vi "UHR-Fleezers Control (host) - 10.8MV_trial.vi"() -> ()   [LabVIEW 2010] (continued)
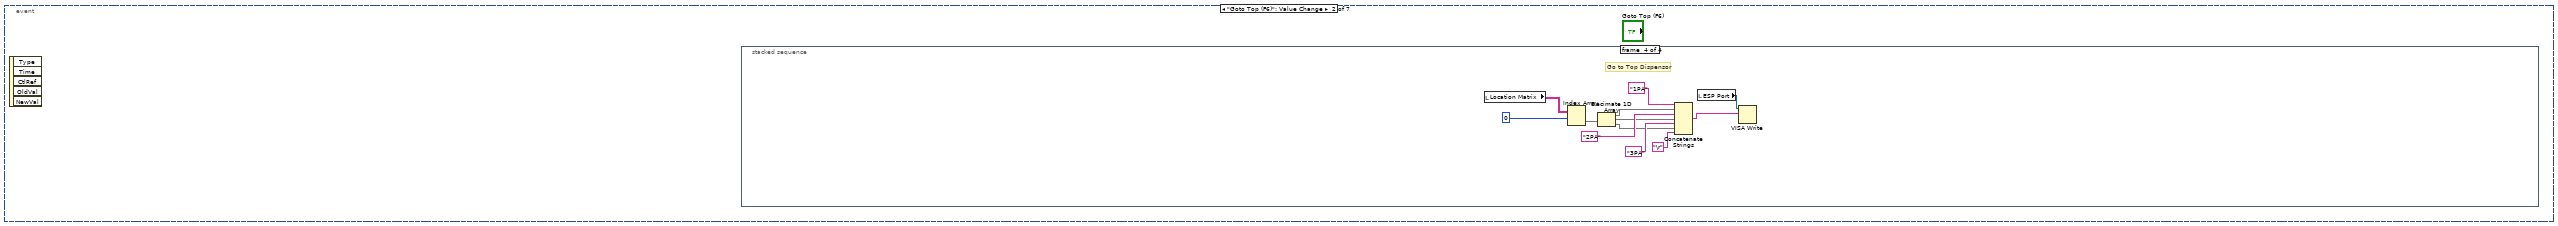
[diagram p3: hidden frame]
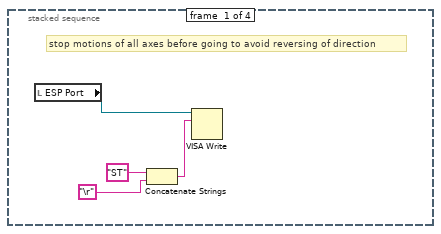
[diagram p4: hidden frame]
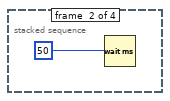
[diagram p5: hidden frame]
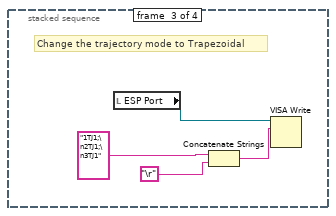
[diagram p6: hidden frame]
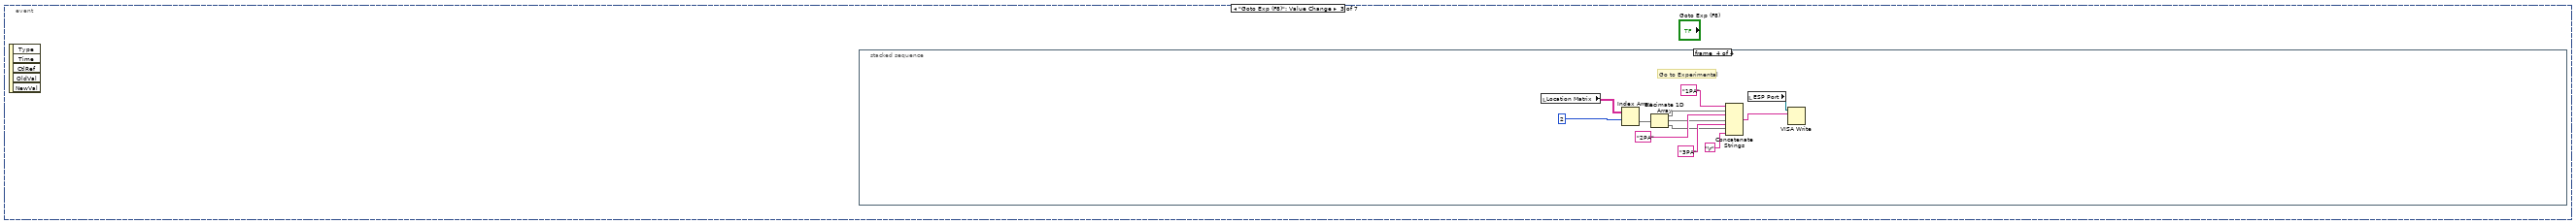
[diagram p7: hidden frame]
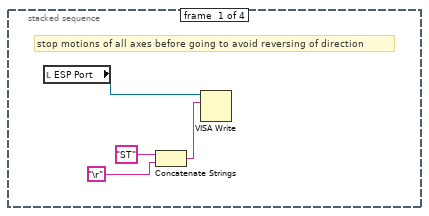
[diagram p8: hidden frame]
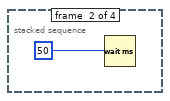
[diagram p9: hidden frame]
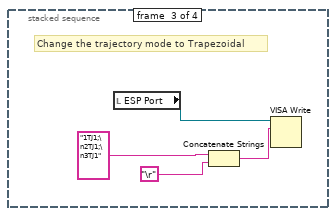
[diagram p10: hidden frame]
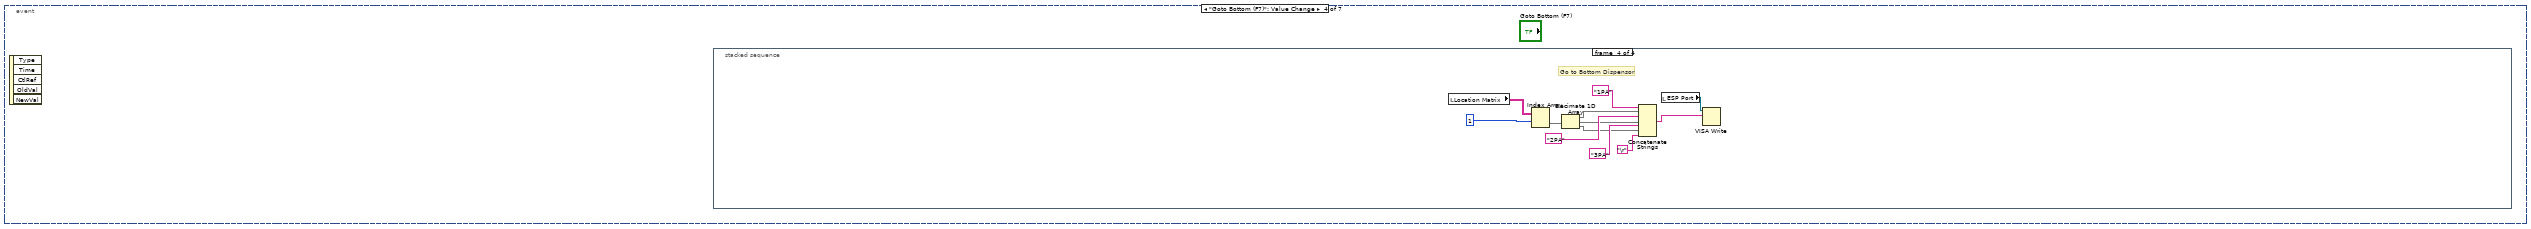
[diagram p11: hidden frame]
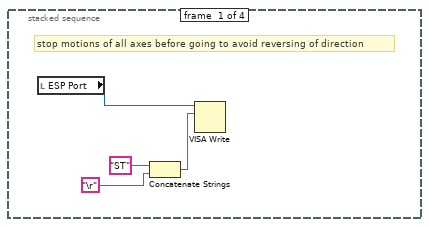
[diagram p12: hidden frame]
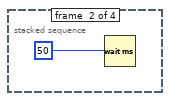
[diagram p13: hidden frame]
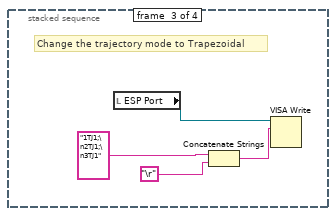
[diagram p14: hidden frame]
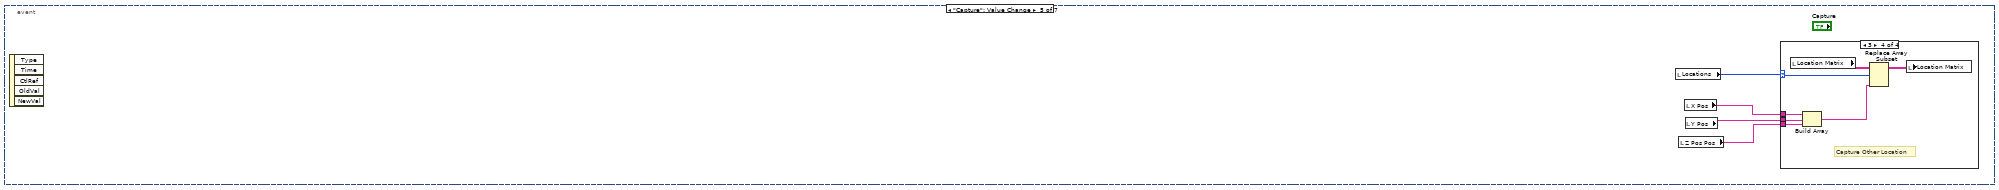
[diagram p15: hidden frame]
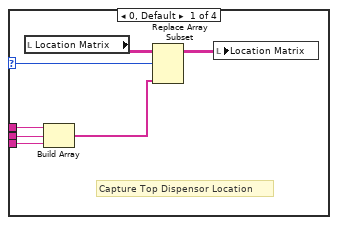
[diagram p16: hidden frame]
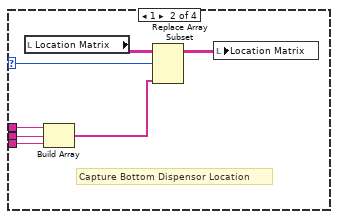
[diagram p17: hidden frame]
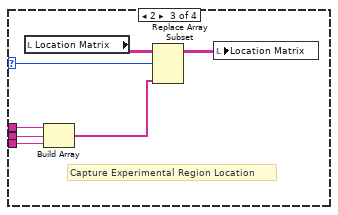
[diagram p18: hidden frame]
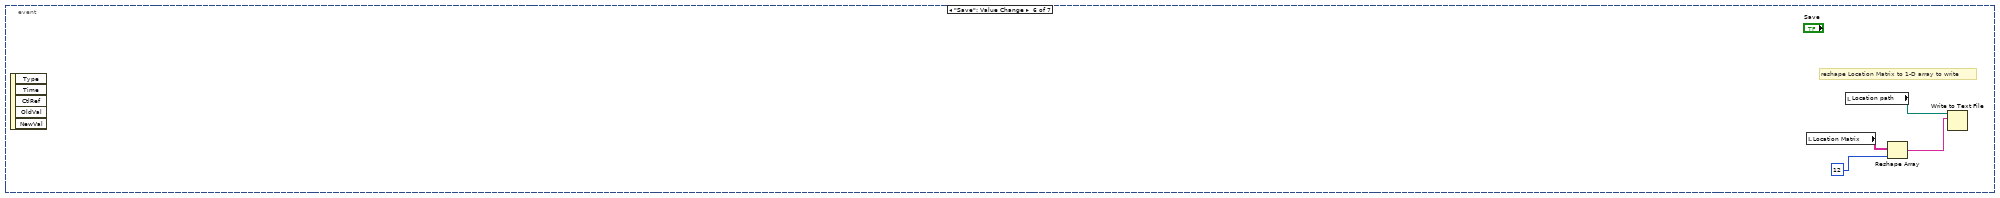
[diagram p19: hidden frame]
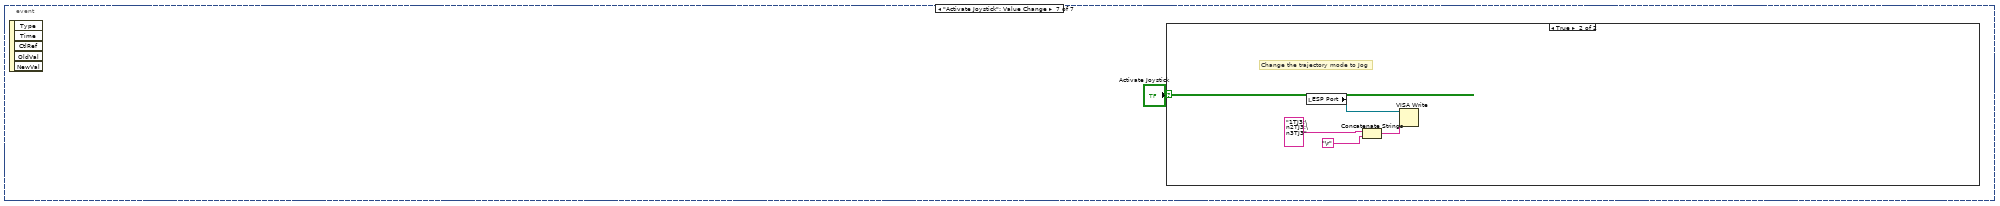
[diagram p20: hidden frame]
                  frame False {
                  }
                  frame True {
                    n1970 = Close File(refnum=w8541) -> ()  [unwired: 1 in, 2 out]
                  }
                }
                n1971 = case shown="True" w8534 {
                  tunnel: w8535 -> [_ w8540]
                  frame False {
                  }
                  frame True {
                    n1972 = Close File(refnum=w8540) -> ()  [unwired: 1 in, 2 out]
                  }
                }
                n1973 = local write "Calibrating Trap..."(w8533) -> ()
                n1974 = call <vilib>:"Beep.vi"() -> ()  [unwired: 3 in, 9 out]
                n1975 = local write "Stop Saving"(w8533) -> ()
                n1976 = property on="Raster Scanning..." class="Bool (strict)"("Val(Sgnl)"=w8533) -> ()  [unwired: 2 in, 2 out]
                "Saving..." <- w8533
              }
              frame True {
                n1977 = local read "Calibrating Trap..."() -> (w8599:bool)
                n1978 = case "Write fl. data" shown="True" w8598 {
                  tunnel: w8597 -> [_ w8633]
                  tunnel: w8596 -> [_ w8632]
                  frame False {
                  }
                  frame True {
                    n1979 = Write to Binary File(file (use dialog)=w8633, data=w8632, 5:FALSE ("prepend array or string size? (T)"), 9:T31."big-endian, network order" ("byte order (0:big-endian, network order)")) -> ()  [unwired: 1 in, 4 out]
                  }
                }
                n1980 = Greater?(x="Save ave N", y=1.0) -> (0:w8602:bool)
                n1981 = Not(x=w8599) -> (.not. x?=w8601:bool)
                n1982 = And(x=w8601, y=w8602) -> (x .and. y?=w8544:bool)
                n1983 = case shown="True" w8544 {
                  tunnel: w8543 -> [w8613 w8624]
                  tunnel: [w8613 w8616] -> w8542
                  tunnel: "Save ave N" -> [_ w8617]
                  frame False {
                  }
                  frame True {
                    w8614 = 2 ("dimension size")
                    n1984 = Array Size(array=w8624) -> (size(s)=w8618:i32)
                    n1985 = Divide(x=w8618, y=w8614) -> (x/y=w8622:dbl)
                    n1986 = Reshape Array(w8624, w8622, w8614) -> (w8623:u64[][])
                    n1987 = Transpose 2D Array(2D array=w8623) -> (transposed array=w8621:u64[][])
                    n1988 = for {
                      tunnel: w8621 -> [w8626] mode=indexing
                      tunnel: [w8625] -> w8615 mode=indexing
                      tunnel: w8617 -> [w8627]
                      workers-P: _ -> [_]
                      n1989 = call "downsample 1D array - U64.vi"("Ave N"=w8627, "Array In"=w8626) -> ("Array Out"=w8625:u64[])  [unwired: 1 in]
                    }
                    n1990 = Transpose 2D Array(2D array=w8615) -> (transposed array=w8620:u64[][])
                    n1991 = Divide(x=w8618, y=w8617) -> (x/y=w8619:dbl)
                    n1992 = Reshape Array(w8620, w8619) -> (w8616:u64[])
                  }
                }
                n1993 = case shown="True" w8544 {
                  tunnel: w8604 -> [w8636 w8648]
                  tunnel: [w8636 w8640] -> w8600
                  tunnel: "Save ave N" -> [_ w8641]
                  tunnel: w8595 -> [_ w8639]
                  frame False {
                    # "don't downsample data for trap calibration"
                  }
                  frame True {
                    n1994 = Array Size(array=w8648) -> (size(s)=w8642:i32)
                    n1995 = Array Size(array=w8639) -> (size(s)=w8638:i32)
                    n1996 = Divide(x=w8642, y=w8638) -> (x/y=w8646:dbl)
                    n1997 = Reshape Array(w8648, w8646, w8638) -> (w8647:i16[][])
                    n1998 = Transpose 2D Array(2D array=w8647) -> (transposed array=w8645:i16[][])
                    n1999 = for {
                      tunnel: w8645 -> [w8651] mode=indexing
                      tunnel: [w8650] -> w8637 mode=indexing
                      tunnel: w8641 -> [w8649]
                      workers-P: _ -> [_]
                      n2000 = call "downsample 1D array - I16.vi"("Ave N"=w8649, "Array In"=w8651) -> ("Array Out"=w8650:i16[])  [unwired: 1 out]
                    }
                    n2001 = Transpose 2D Array(2D array=w8637) -> (transposed array=w8644:i16[][])
                    n2002 = Divide(x=w8642, y=w8641) -> (x/y=w8643:dbl)
                    n2003 = Reshape Array(w8644, w8643) -> (w8640:i16[])
                  }
                }
                n2004 = Index Array(array=w8566, index=1) -> (element=w8569:waveform(dbl))
                n2005 = Index Array(array=w8566, index=0) -> (element=w8571:waveform(dbl))
                n2006 = Unbundle By Name(w8569) -> ("Y"=w8573:dbl[])
                n2007 = Unbundle By Name(w8571) -> ("Y"=w8581:dbl[])
                n2008 = case "Write trap pos. data" shown="True" w8547 {
                  tunnel: w8546 -> [_ w8629]
                  tunnel: w8542 -> [_ w8628]
                  frame False {
                  }
                  frame True {
                    n2009 = Write to Binary File(file (use dialog)=w8629, data=w8628, 5:FALSE ("prepend array or string size? (T)"), 9:T31."big-endian, network order" ("byte order (0:big-endian, network order)")) -> ()  [unwired: 1 in, 4 out]
                  }
                }
                n2010 = Write to Binary File(file (use dialog)=w8607, data=w8600, 5:FALSE ("prepend array or string size? (T)"), 9:T31."big-endian, network order" ("byte order (0:big-endian, network order)")) -> ()  [unwired: 1 in, 4 out]
                n2011 = feedback #26(w8573) -> (w8575:dbl[])
                n2012 = Build Array (concatenate)(w8575, w8573) -> (w8574:dbl[])
                n2013 = Select(t=w8573, s=w8549, f=w8574) -> (s? t:f=w8559:dbl[])
                n2014 = feedback-in #26(w8559) -> ()
                n2015 = feedback #27(w8581) -> (w8594:dbl[])
                n2016 = Build Array (concatenate)(w8594, w8581) -> (w8593:dbl[])
                n2017 = Select(t=w8581, s=w8549, f=w8593) -> (s? t:f=w8568:dbl[])
                n2018 = feedback-in #27(w8568) -> ()
                n2019 = Divide(x=w8608, y=w8609) -> (x/y=w8611:dbl)
                n2020 = Multiply(x=w8611, y=100.0) -> (x*y=w8610:dbl)
                n2021 = Build Array(w8568, w8559) -> (→"Saved APD":dbl[][])
                n2022 = Array Size(array=w8568) -> (size(s)=w8586:i32)
                n2023 = Unbundle By Name(w8588) -> ("Y"=w8592:dbl[])
                n2024 = Subtract(x=w8586, y="N pts to average") -> (x-y=w8562:i32)
                n2025 = Multiply(x="N pts to average", y=u16 2) -> (x*y=w8563:u16)
                n2026 = Subtract(x=w8586, y=w8563) -> (x-y=w8561:i32)
                n2027 = feedback #28(w8592) -> (w8591:dbl[])
                n2028 = Build Array (concatenate)(w8591, w8592) -> (w8590:dbl[])
                n2029 = Select(t=w8592, s=w8549, f=w8590) -> (s? t:f=w8589:dbl[])
                "Trap Delta Graph" <- w8589
                n2030 = feedback-in #28(w8589) -> ()
                n2031 = Array Subset(array=w8568, index=w8562, length="N pts to average") -> (w8585:dbl[])
                n2032 = Array Subset(array=w8568, index=w8561, length="N pts to average") -> (w8584:dbl[])
                n2033 = Array Subset(array=w8559, index=w8562, length="N pts to average") -> (w8565:dbl[])
                n2034 = Array Subset(array=w8559, index=w8561, length="N pts to average") -> (w8564:dbl[])
                n2035 = call <vilib>:"Mean.vi"("X"=w8585) -> ("mean"=w8583:dbl)  [unwired: 1 out]
                n2036 = call <vilib>:"Mean.vi"("X"=w8565) -> ("mean"=w8558:dbl)  [unwired: 1 out]
                n2037 = call <vilib>:"Mean.vi"("X"=w8584) -> ("mean"=w8582:dbl)  [unwired: 1 out]
                n2038 = call <vilib>:"Mean.vi"("X"=w8564) -> ("mean"=w8557:dbl)  [unwired: 1 out]
                n2039 = Subtract(x=w8558, y=w8557) -> (x-y=w8548:dbl)
                "Delta Fl. 2" <- w8548
                n2040 = Subtract(x=w8583, y=w8582) -> (x-y=w8580:dbl)
                "Delta Fl. 1" <- w8580
                n2041 = Initialize Array(w8580, 1 ("dimension size")) -> (w8577:dbl[])
                n2042 = Initialize Array(w8548, 1 ("dimension size")) -> (w8554:dbl[])
                n2043 = feedback #29(w8577) -> (w8578:dbl[])
                n2044 = Build Array (concatenate)(w8578, w8577) -> (w8576:dbl[])
                n2045 = feedback #30(w8554) -> (w8555:dbl[])
                n2046 = Build Array (concatenate)(w8555, w8554) -> (w8553:dbl[])
                n2047 = Select(t=w8577, s=w8549, f=w8576) -> (s? t:f=w8552:dbl[])
                n2048 = feedback-in #29(w8552) -> ()
                n2049 = Select(t=w8554, s=w8549, f=w8553) -> (s? t:f=w8551:dbl[])
                n2050 = feedback-in #30(w8551) -> ()
                n2051 = Build Array(w8552, w8551) -> (→"Save APD Deriv":dbl[][])
              }
            }
            "Progress" <- w8525
            "Progress 2" <- w8525
          }
        }
      }
    }
    n2052 = Bundle By Name(cluster=w5568, "Green FB Ch 0"=w5567, "Green FB Ch 1"=w5566) -> (w5546:T50)
    "Green FB Signals (V)" <- w5546
    n2053 = Unbundle By Name(w5546) -> ("Green FB Ch 2"=→"Green FB Plot":dbl)
    n2054 = local read "wait to reset values"() -> (w5638:bool)
    n2055 = Not(x=w5635) -> (.not. x?=w5639:bool)
    n2056 = And(x=w5639, y=w5638) -> (x .and. y?=w5640:bool)
    n2057 = case "Part of MCL raster scanning: returns to initial positions after scan done" shown="True" w5640 {
      tunnel: w5643 -> [w7242 w7249]
      tunnel: [w7242 w7248] -> w5642
      tunnel: w5637 -> [w7241 w7247]
      tunnel: [w7241 w7246] -> w5636
      frame False {
      }
      frame True {
        w7257 = 10.0 ("y")
        w7256 = 32767.0 ("y")
        # "to return scan values\nafter a synchronous \nAOM scan"
        n2058 = local read "AO2"() -> (w7250:dbl)
        n2059 = local read "AO1"() -> (w7251:dbl)
        n2060 = local write "wait to reset values"(FALSE ("wait to reset values")) -> ()
        n2061 = Multiply(x=w7251, y=w7256) -> (x*y=w7253:dbl)
        n2062 = Multiply(x=w7250, y=w7256) -> (x*y=w7255:dbl)
        n2063 = Divide(x=w7253, y=w7257) -> (x/y=w7252:dbl)
        n2064 = Divide(x=w7255, y=w7257) -> (x/y=w7254:dbl)
        n2065 = To Word Integer(number=w7252) -> (16bit integer=w7258:i16)
        n2066 = To Word Integer(number=w7254) -> (16bit integer=w7259:i16)
        n2067 = local read "Total Counts (ticks)"() -> (w7243:u32)
        n2068 = xnode "Read/Write Control"("FPGA VI Reference In"=w7249, "error in"=w7247, "AO1"=w7258, "AO2"=w7259, "MCL count"=w7243) -> ("FPGA VI Reference Out"=w7248:T19, "error out"=w7246:errorcluster)
        n2069 = local read "Scan Range (V)\n(of steps)"() -> (w7244:dbl)
        n2070 = property on="Scan Range (V)\n(of steps)" class="DigNum (strict)"("Val(Sgnl)"=w7244) -> ()  [unwired: 2 in, 2 out]
      }
    }
    n2071 = node-c288() -> ()  [unwired: 2 out]
  }
  n2072 = node-c288(3 ("Processor")) -> (w74:T26)  [unwired: 3 out]
  n2073 = timed-loop "Oscillate AOD (debugging)" {
    tunnel: w24 -> [w8653]
    tunnel: [w8652] -> w36
    timing: w74 -> [_]
    timing-out: [_] -> w73
    stop <- w8652 stop-if-true
    n2074 = node-c288() -> ()  [unwired: 2 out]
    n2075 = event shown="[0] \"Oscillate Set 2\", \"Fish for Tether\": Value Change" {
      selector: _ -> [_ _ _]
      dyn-events: _ -> [_ _ _]
      timeout: _ -> [_ _ _]
      tunnel: w8653 -> [w8660 _ _]
      tunnel: [FALSE ("Stop All") _ w8928] -> w8652
      event "Oscillate Set 2", "Fish for Tether": Value Change {
        n2076 = event-data() -> ()  [unwired: 6 out]
        n2077 = local read "Oscillate Set 2"() -> (w8659:bool)
        n2078 = Or(x=w8659, y="Fish for Tether") -> (x .or. y?=w8657:bool)
        n2079 = case shown="True" w8657 {
          tunnel: w8660 -> [_ w8663]
          tunnel: "Fish for Tether" -> [_ w8662]
          frame False {
          }
          frame True {
            n2080 = case shown="True" w8662 {
              frame False {
              }
              frame True {
                n2081 = local write "Scan axis 2"(TRUE) -> ()
                n2082 = local write "Tether"(FALSE ("Tether")) -> ()
              }
            }
            n2083 = node-c288("Period") -> (w8665:T26)  [unwired: 3 out]
            n2084 = timed-loop "Oscillate AOD" {
              timing: w8665 -> [_]
              timing-out: [_] -> w8664
              tunnel: w8663 -> [w8675]
              tunnel: w8662 -> [w8674]
              i -> [w8677]
              stop <- w8673 stop-if-true
              n2085 = node-c288() -> (w8676:i64)  [unwired: 1 out]
              n2086 = flat-sequence {
                tunnel: w8677 -> [w8703]
                tunnel: w8676 -> [w8702]
                tunnel: w8675 -> [w8686]
                tunnel: w8674 -> [w8688]
                tunnel: [w8688] -> w8672
                tunnel: [w8687] -> w8671
                tunnel: [w8685] -> w8670
                tunnel: [w8682] -> w8668
                tunnel: w8672 -> [w8739]
                tunnel: w8671 -> [w8737]
                tunnel: w8670 -> [w8736]
                tunnel: [w8735] -> w8669
                tunnel: w8668 -> [w8734]
                tunnel: [w8803] -> w8673
                tunnel: w8669 -> [w8801]
                frame #0 {
                  n2087 = Divide(x=w8702, y=i64 1000) -> (x/y=w8697:dbl)
                  n2088 = Multiply(x=w8697, y=w8703) -> (x*y=w8699:dbl)
                  n2089 = Multiply(x="Osc. freq. (Hz)", y=6.283185307179586) -> (x*y=w8700:dbl)
                  n2090 = Multiply(x=w8700, y=w8699) -> (x*y=w8684:dbl)
                  n2091 = local read "BD 1 Frequency 2 (MHz)"() -> (w8681:dbl)
                  n2092 = local read "BD 1 Frequency 1 (MHz)"() -> (w8678:dbl)
                  n2093 = case shown="True" w8688 {
                    tunnel: w8684 -> [w8709 w8716]
                    tunnel: w8681 -> [_ w8726]
                    tunnel: [w8706 w8710] -> w8689
                    tunnel: [FALSE w8719] -> w8685
                    tunnel: [0.0 w8712] -> w8682
                    tunnel: w8678 -> [_ w8711]
                    frame False {
                      n2094 = Sine(x=w8709) -> (sin(x)=w8707:dbl)
                      n2095 = Multiply(x=w8707, y="Osc. amp. (MHz)") -> (x*y=w8706:dbl)
                    }
                    frame True {
                      n2096 = Cosine(x=w8716) -> (cos(x)=w8729:dbl)
                      n2097 = Subtract(x=w8726, y=w8711) -> (x-y=w8725:dbl)
                      n2098 = Decrement(x=w8729) -> (x-1=w8728:dbl)
                      n2099 = Subtract(x=w8725, y="Closest Delta (MHz)") -> (x-y=w8722:dbl)
                      n2100 = Divide(x=w8728, y=2.0) -> (x/y=w8723:dbl)
                      n2101 = Multiply(x=w8723, y=w8722) -> (x*y=w8710:dbl)
                      n2102 = local read "Vec Mean of T1 T2"() -> (w8718:dbl[])
                      n2103 = Greater?(x=w8718, y="Stop F (pN)") -> (0:w8720:bool[])
                      n2104 = Or Array Elements(Boolean array=w8720) -> (logical OR=w8719:bool)
                      n2105 = Divide(x=w8716, y=6.283185307179586) -> (x/y=w8715:dbl)
                      n2106 = Round Toward +Infinity(x=w8715) -> (ceil(x): smallest int >= x=w8712:dbl)
                      "Attempts" <- w8712
                      n2107 = Greater?(x=w8712, y="Attempt Limit") -> (0:w8714:bool)
                      n2108 = case shown="True" w8714 {
                        frame False {
                        }
                        frame True {
                          n2109 = local write "Fish for Tether"(FALSE ("Fish for Tether")) -> ()
                          n2110 = call <vilib>:"Beep.vi"() -> ()  [unwired: 3 in, 9 out]
                          n2111 = local read "Messages"() -> (w8731:string)
                          n2112 = call "Update messages.vi"("Message to add"="Tether fishing timeout." ("Messages"), "Old message string"=w8731) -> ("New message string"=→"Messages":string)
                        }
                      }
                    }
                  }
                  n2113 = local read "Y RF Frequency Limits (MHz)"() -> (w8690:T16)
                  n2114 = local read "X RF Frequency Limits (MHz)"() -> (w8691:T16)
                  n2115 = local read "BD 1 Frequency 3 (MHz)"() -> (w8696:dbl)
                  n2116 = local read "BD 2 Frequency 2 (MHz)"() -> (w8680:dbl)
                  n2117 = Select(t=w8681, s="Scan axis 2", f=w8680) -> (s? t:f=w8692:dbl)
                  n2118 = Add(x=w8689, y=w8692) -> (x+y=w8687:dbl)
                  n2119 = Select(t=w8687, s="Scan axis 2", f=w8681) -> (s? t:f=w8679:dbl)
                  n2120 = Select(t=w8680, s="Scan axis 2", f=w8687) -> (s? t:f=w8694:dbl)
                  n2121 = local read "BD 2 Frequency 3 (MHz)"() -> (w8695:dbl)
                  n2122 = call "set RF board frequency - interlace.vi"("Board 2 Frequency Limits"=w8690, "Board 1 Frequency Limits"=w8691, "FPGA VI Reference In"=w8686, "Board 2 Frequency 3 (MHz)"=w8695, "Board 1 Frequency 3 (MHz)"=w8696, "Board 2 Frequency 2 (MHz)"=w8680, "Board 2 Frequency 1 (MHz)"=w8694, "Board 1 Frequency 2 (MHz)"=w8679, "Board 1 Frequency 1  (MHz)"=w8678) -> ()  [unwired: 1 in, 2 out]
                }
                frame #1 {
                  n2123 = And(x=w8739, y=w8736) -> (x .and. y?=w8738:bool)
                  n2124 = case "Only if were fishing and now formed tether" shown="True" w8738 {
                    tunnel: w8737 -> [w8741 w8753]
                    tunnel: [w8740 w8752] -> w8735
                    tunnel: w8734 -> [_ w8748]
                    frame False {
                      n2125 = local read "Fish for Tether"() -> (w8740:bool)
                      n2126 = case shown="True" w8740 {
                        tunnel: w8741 -> [_ _]
                        frame False {
                        }
                        frame True {
                        }
                      }
                    }
                    frame True {
                      w8752 = FALSE ("Fish for Tether")
                      n2127 = call <vilib>:"Beep.vi"() -> ()  [unwired: 3 in, 9 out]
                      n2128 = Number To Decimal String(number=w8748, width (-)=i16 1) -> (decimal integer string=w8746:string)
                      n2129 = case shown="\"2\", \"3\", \"4\", \"5\", \"6\"" "Then..." {
                        selector: "Then..." -> [_ w8756]
                        tunnel: w8753 -> [w8755 _]
                        frame "1", Default {
                          # "do nothing"
                          n2130 = property on="BD 1 Frequency 1 (MHz)" class="DigNum (strict)"("Val(Sgnl)"=w8755) -> ()  [unwired: 2 in, 2 out]
                        }
                        frame "2", "3", "4", "5", "6" {
                          n2131 = flat-sequence {
                            tunnel: w8756 -> [w8758]
                            frame #0 {
                              n2132 = property on="Trap Delta (MHz)" class="DigNum (strict)"("Val(Sgnl)"="Move to Delta 1 (MHz)") -> ()  [unwired: 2 in, 2 out]
                            }
                            frame #1 {
                              n2133 = case shown="\"5\", \"6\"" w8758 {
                                selector: w8758 -> [w8761 w8771 _]
                                frame "3", "4" {
                                n2134 = flat-sequence {
                                tunnel: w8761 -> [w8762]
                                tunnel: [w8762] -> w8759
                                tunnel: [w8764] -> w8760
                                tunnel: w8759 -> [w8764]
                                tunnel: w8760 -> [w8768]
                                frame #0 {
                                n2135 = property on="Green Laser ON/Interlacing" class="Bool (strict)"("Val(Sgnl)"=TRUE ("Value (Signaling)")) -> ()  [unwired: 2 in, 2 out]
                                }
                                frame #1 {
                                n2136 = Multiply(x="Wait Before Save (s)", y=u32 1000 ("x")) -> (x*y=w8766:u32)
                                n2137 = Wait (ms)(milliseconds to wait=w8766) -> ()  [unwired: 1 out]
                                }
                                frame #2 {
                                n2138 = property on="Start Saving" class="Bool (strict)"("Value"=TRUE ("Start Saving")) -> ()  [unwired: 2 in, 2 out]
                                n2139 = case shown="Default" w8768 {
                                frame Default {
                                }
                                frame "4" {
                                n2140 = property on="Fl. Triggered..." class="Bool (strict)"("Val(Sgnl)"=TRUE ("Value (Signaling)")) -> ()  [unwired: 2 in, 2 out]
                                }
                                }
                                }
                                }
                                }
                                frame "5", "6" {
                                n2141 = stacked-sequence {
                                tunnel: w8771 -> [_ _ _ _ _ _ _ _ w8788 _ _]
                                frame #0 {
                                n2142 = Replace Array Subset(array=u32[] [0] ("Index Values"), new element="Raster Set Upon Tether", index=0) -> (w8772:u32[])
                                n2143 = property on="Saved AOD Raster Scan Parameter Sets" class="Arr (strict)"("Index Values"=w8772) -> ()  [unwired: 2 in, 2 out]
                                }
                                frame #1 {
                                n2144 = Wait (ms)(milliseconds to wait=u32 500) -> ()  [unwired: 1 out]
                                }
                                frame #2 {
                                n2145 = property on="Load parameters" class="Bool (strict)"("Val(Sgnl)"=TRUE ("Value (Signaling)")) -> ()  [unwired: 2 in, 2 out]
                                }
                                frame #3 {
                                n2146 = Wait (ms)(milliseconds to wait=u32 500) -> ()  [unwired: 1 out]
                                }
                                frame #4 {
                                n2147 = property on="Trap Raster Scan" class="Bool (strict)"("Val(Sgnl)"=TRUE ("Value (Signaling)")) -> ()  [unwired: 2 in, 2 out]
                                }
                                frame #5 {
                                n2148 = Wait (ms)(milliseconds to wait=u32 2000) -> ()  [unwired: 1 out]
                                }
                                frame #6 {
                                n2149 = while {
                                stop <- w8783 stop-if-true
                                n2150 = local read "Raster Scanning..."() -> (w8782:bool)
                                n2151 = local read "Saving..."() -> (w8785:bool)
                                n2152 = Wait (ms)(milliseconds to wait=u32 100) -> ()  [unwired: 1 out]
                                n2153 = Not(x=w8785) -> (.not. x?=w8784:bool)
                                n2154 = Not(x=w8782) -> (.not. x?=w8781:bool)
                                n2155 = And(x=w8784, y=w8781) -> (x .and. y?=w8783:bool)
                                }
                                }
                                frame #7 {
                                n2156 = property on="Trap Delta (MHz)" class="DigNum (strict)"("Val(Sgnl)"="Move to Delta 2 (MHz)") -> ()  [unwired: 2 in, 2 out]
                                }
                                frame #8 {
                                n2157 = local read "Tether"() -> (w8789:bool)
                                n2158 = case shown="True" w8789 {
                                tunnel: w8788 -> [_ w8790]
                                frame False {
                                }
                                frame True {
                                n2159 = flat-sequence {
                                tunnel: w8790 -> [w8792]
                                frame #0 {
                                n2160 = Wait (ms)(milliseconds to wait=u32 500) -> ()  [unwired: 1 out]
                                }
                                frame #1 {
                                n2161 = case shown="\"6\"" w8792 {
                                frame Default {
                                }
                                frame "6" {
                                n2162 = property on="Green Laser ON/Interlacing" class="Bool (strict)"("Val(Sgnl)"=TRUE ("Green Laser ON/Interlacing")) -> ()  [unwired: 2 in, 2 out]
                                }
                                }
                                }
                                frame #2 {
                                n2163 = Wait (ms)(milliseconds to wait=u32 500) -> ()  [unwired: 1 out]
                                }
                                frame #3 {
                                n2164 = local write "Start Saving"("Save at end (5, 6)") -> ()
                                }
                                }
                                }
                                }
                                }
                                frame #9 {
                                n2165 = local read "Bead Sep. Int. Time (s)"() -> (w8798:dbl)
                                n2166 = Multiply(x=w8798, y=1000.0) -> (x*y=w8797:dbl)
                                n2167 = Wait (ms)(milliseconds to wait=w8797) -> ()  [unwired: 1 out]
                                }
                                frame #10 {
                                n2168 = property on="Rescale on Mean" class="Bool (strict)"("Val(Sgnl)"=TRUE ("Value (Signaling)")) -> ()  [unwired: 2 in, 2 out]
                                }
                                }
                                }
                                frame "2", Default {
                                }
                              }
                            }
                          }
                        }
                      }
                      n2169 = Concatenate Strings("Formed tether in ", w8746, " attempt(s)." ("string")) -> (w8743:string)
                      n2170 = local read "Messages"() -> (w8750:string)
                      n2171 = local write "Fish for Tether"(w8752) -> ()
                      n2172 = call "Update messages.vi"("Message to add"=w8743, "Old message string"=w8750) -> ("New message string"=w8749:string)
                      n2173 = local write "Messages"(w8749) -> ()
                      n2174 = Get Date/Time In Seconds() -> (seconds since 1Jan1904=→"Time tether formed":timestamp)
                      "Tether" <- "Tether Alarm?"
                    }
                  }
                }
                frame #2 {
                  n2175 = local read "Oscillate Set 2"() -> (w8802:bool)
                  n2176 = local read "Stop All"() -> (w8804:bool)
                  n2177 = Not Or(1:w8801, 2:w8802) -> (0:w8800:bool)
                  n2178 = Compound Arithmetic op=OR(w8804, w8800) -> (w8803:bool)
                }
              }
              n2179 = node-c288() -> ()  [unwired: 2 out]
            }
            n2180 = node-c288(w8664) -> ()  [unwired: 1 out]
          }
        }
      }
      event "Fl. Triggered...": Value Change {
        n2181 = event-data() -> ()  [unwired: 7 out]
        n2182 = case shown="True" "Fl. Triggered..." {
          frame False {
          }
          frame True {
            n2183 = node-c288() -> (w8816:T26)  [unwired: 4 out]
            n2184 = timed-loop {
              timing: w8816 -> [_]
              timing-out: [_] -> w8815
              tunnel: "Action" -> [w8820]
              shift-right: [w8817] -> _
              shift-left: u8 255 -> [w8819]
              stop <- w8821 stop-if-true
              n2185 = node-c288() -> ()  [unwired: 2 out]
              n2186 = flat-sequence {
                tunnel: w8820 -> [w8833]
                tunnel: w8819 -> [w8830]
                tunnel: [w8829] -> w8818
                tunnel: [w8919] -> w8821
                tunnel: w8818 -> [w8918]
                tunnel: [w8918] -> w8817
                frame #0 {
                  n2187 = local read "Delta Fl. 2"() -> (w8824:dbl)
                  n2188 = local read "Delta Fl. 1"() -> (w8825:dbl)
                  n2189 = Select(t=w8825, s="APD to Watch", f=w8824) -> (s? t:f=w8823:dbl)
                  n2190 = Multiply(x="Fl. Delta Thresh. (kHz)", y=1000.0) -> (x*y=w8832:dbl)
                  n2191 = Greater?(x=w8823, y=w8832) -> (0:w8827:bool)
                  n2192 = Or(x="Force Yank", y=w8827) -> (x .or. y?=w8828:bool)
                  n2193 = case shown="True" w8828 {
                    tunnel: w8833 -> [_ w8843]
                    tunnel: w8830 -> [w8835 w8839]
                    tunnel: [w8835 w8836] -> w8829
                    frame False {
                    }
                    frame True {
                      n2194 = flat-sequence {
                        tunnel: w8840 -> [w8849]
                        tunnel: [w8849] -> w8844
                        tunnel: w8843 -> [w8848]
                        tunnel: [w8848] -> w8842
                        tunnel: [w8847] -> w8841
                        tunnel: w8839 -> [w8846]
                        tunnel: [w8845] -> w8838
                        tunnel: w8844 -> [w8874]
                        tunnel: w8842 -> [w8873]
                        tunnel: w8841 -> [w8872]
                        tunnel: w8838 -> [w8871]
                        tunnel: [w8871] -> w8837
                        tunnel: w8837 -> [w8916]
                        tunnel: [w8916] -> w8836
                        frame #0 {
                          n2195 = call <vilib>:"Beep.vi"() -> ()  [unwired: 3 in, 9 out]
                          n2196 = local write "Waiting"(FALSE ("Waiting")) -> ()
                          n2197 = Increment(x=w8846) -> (x+1=w8845:u8)
                          n2198 = case shown="\"Yank\"" w8848 {
                            tunnel: w8845 -> [_ _ w8855]
                            frame "Image" {
                              n2199 = property on="Confocal Image" class="Bool (strict)"("Val(Sgnl)"=TRUE ("Value (Signaling)")) -> ()  [unwired: 2 in, 2 out]
                            }
                            frame "Alarm", Default {
                            }
                            frame "Yank" {
                              n2200 = flat-sequence {
                                tunnel: w8855 -> [w8858]
                                tunnel: [w8857] -> w8854
                                tunnel: ["N Array El"] -> w8853
                                tunnel: w8854 -> [w8868]
                                tunnel: w8853 -> [w8864]
                                frame #0 {
                                n2201 = Multiply(x="Yank Delay (s)", y=1000.0) -> (x*y=w8861:dbl)
                                n2202 = Quotient & Remainder(x=w8858, y="N Array El") -> (x-y*floor(x/y)=w8857:u8)  [unwired: 1 out]
                                n2203 = Wait (ms)(milliseconds to wait=w8861) -> ()  [unwired: 1 out]
                                }
                                frame #1 {
                                n2204 = Random Number (0-1)() -> (number: 0 to 1=w8865:dbl)
                                n2205 = Multiply(x=w8864, y=w8865) -> (x*y=w8863:dbl)
                                n2206 = Round Toward -Infinity(1:w8863) -> (0:w8862:dbl)
                                n2207 = Select(t=w8862, s="Random Choice", f=w8868) -> (s? t:f=w8866:dbl)
                                n2208 = Index Array(array="Yank to Delta Array (MHz)", index=w8866) -> (element=w8869:dbl)
                                n2209 = property on="Trap Delta (MHz)" class="DigNum (strict)"("Val(Sgnl)"=w8869) -> ()  [unwired: 2 in, 2 out]
                                }
                              }
                            }
                          }
                          n2210 = local read "Time (s)"() -> (w8847:dbl)
                          "Fl. High" <- TRUE ("Yanking")
                        }
                        frame #1 {
                          n2211 = node-c288() -> (w8876:T26)  [unwired: 4 out]
                          n2212 = timed-loop {
                            timing: w8876 -> [_]
                            timing-out: [_] -> w8875
                            tunnel: w8874 -> [w8892]
                            tunnel: w8873 -> [w8890]
                            tunnel: w8872 -> [w8889]
                            stop <- w8891 stop-if-true
                            n2213 = node-c288() -> ()  [unwired: 2 out]
                            n2214 = local read "Fl. Delta Thresh. (kHz)"() -> (w8884:dbl)
                            n2215 = local read "Fl. Triggered..."() -> (w8893:bool)
                            n2216 = local read "Delta Fl. 1"() -> (w8880:dbl)
                            n2217 = local read "Delta Fl. 2"() -> (w8878:dbl)
                            n2218 = local read "Stop All"() -> (w8887:bool)
                            n2219 = local read "APD to Watch"() -> (w8879:bool)
                            n2220 = Select(t=w8880, s=w8879, f=w8878) -> (s? t:f=w8877:dbl)
                            n2221 = Not(x=w8893) -> (.not. x?=w8888:bool)
                            n2222 = Multiply(x=w8884, y=1000.0) -> (x*y=w8883:dbl)
                            n2223 = Negate(x=w8883) -> (-x=w8882:dbl)
                            n2224 = Less?(x=w8877, y=w8882) -> (x < y?=w8886:bool)
                            n2225 = Compound Arithmetic op=OR(w8886, w8887, w8888, "Force Reset") -> (w8891:bool)
                            n2226 = case shown="True" w8891 {
                              tunnel: w8892 -> [_ w8904]
                              tunnel: w8890 -> [_ w8903]
                              tunnel: w8889 -> [_ w8901]
                              frame False {
                              }
                              frame True {
                                n2227 = case shown="\"Yank\"" w8903 {
                                tunnel: w8904 -> [_ w8905]
                                frame "Image", Default {
                                }
                                frame "Yank" {
                                n2228 = flat-sequence {
                                tunnel: [w8910] -> w8906
                                tunnel: w8905 -> [w8910]
                                tunnel: w8906 -> [w8911]
                                frame #0 {
                                n2229 = local read "Yank Delay (s)"() -> (w8909:dbl)
                                n2230 = Multiply(x=w8909, y=1000.0) -> (x*y=w8907:dbl)
                                n2231 = Wait (ms)(milliseconds to wait=w8907) -> ()  [unwired: 1 out]
                                }
                                frame #1 {
                                n2232 = property on="Trap Delta (MHz)" class="DigNum (strict)"("Val(Sgnl)"=w8911) -> ()  [unwired: 2 in, 2 out]
                                }
                                }
                                }
                                }
                                n2233 = local read "Time (s)"() -> (w8902:dbl)
                                n2234 = Subtract(x=w8902, y=w8901) -> (x-y=w8898:dbl)
                                "Duration (s)" <- w8898
                                n2235 = Number To Decimal String(number=w8898, width (-)=i16 0) -> (decimal integer string=w8896:string)
                                n2236 = Concatenate Strings(w8896, " s fluorescence event." ("string")) -> (w8894:string)
                                n2237 = local read "Messages"() -> (w8900:string)
                                n2238 = call "Update messages.vi"("Message to add"=w8894, "Old message string"=w8900) -> ("New message string"=w8899:string)
                                n2239 = call <vilib>:"Beep.vi"() -> ()  [unwired: 3 in, 9 out]
                                n2240 = local write "Messages"(w8899) -> ()
                              }
                            }
                            n2241 = node-c288() -> ()  [unwired: 2 out]
                          }
                          n2242 = node-c288(w8875) -> ()  [unwired: 1 out]
                        }
                        frame #2 {
                          n2243 = local write "Fl. High"(FALSE ("Yanking")) -> ()
                        }
                      }
                      n2244 = local read "Trap Delta (MHz)"() -> (w8840:dbl)
                    }
                  }
                }
                frame #1 {
                  n2245 = local read "Stop All"() -> (w8922:bool)
                  n2246 = local read "Fl. Triggered..."() -> (w8920:bool)
                  n2247 = Not(x=w8920) -> (.not. x?=w8921:bool)
                  n2248 = Or(x=w8921, y=w8922) -> (x .or. y?=w8919:bool)
                  n2249 = Not(x=w8919) -> (.not. x?=→"Waiting":bool)
                }
              }
              n2250 = node-c288() -> ()  [unwired: 2 out]
            }
            n2251 = node-c288(w8815) -> ()  [unwired: 1 out]
          }
        }
      }
      event "Stop All": Value Change {
        n2252 = event-data() -> ()  [unwired: 7 out]
        n2253 = local read "Stop All"() -> (w8928:bool)
      }
    }
    n2254 = node-c288() -> ()  [unwired: 2 out]
  }
  n2255 = node-c288(w14) -> ()  [unwired: 1 out]
  n2256 = node-c288(w68) -> ()  [unwired: 1 out]
  n2257 = node-c288(w75) -> ()  [unwired: 1 out]
  n2258 = node-c288(w73) -> ()  [unwired: 1 out]
  n2259 = node-c288(w163) -> ()  [unwired: 1 out]
  n2260 = flat-sequence {
    tunnel: w33 -> [w8933]
    tunnel: [w8932] -> w39
    tunnel: [w8929] -> w38
    tunnel: w37 -> [_]
    tunnel: w36 -> [_]
    tunnel: w35 -> [_]
    tunnel: w34 -> [_]
    tunnel: w32 -> [w8930]
    tunnel: w39 -> [w8995]
    tunnel: w38 -> [w8994]
    frame #0 {
      w8931 = FALSE ("APD to FIFO")
      n2261 = xnode "Read/Write Control"("FPGA VI Reference In"=w8933, "error in"=w8930, "APD to FIFO"=w8931, "AI to FIFO"=w8931) -> ("FPGA VI Reference Out"=w8932:T19, "error out"=w8929:errorcluster)
    }
    frame #1 {
      n2262 = xnode "Invoke Method"("FPGA VI Reference In"=w8995, "error in"=w8994) -> ("FPGA VI Reference Out"=w8993:T19)  [unwired: 1 out]
      n2263 = xnode "Close FPGA VI Reference"("FPGA VI Reference In"=w8993) -> ()  [unwired: 1 in, 1 out]
    }
  }
